vi "HFRR ADV v037.vi"() -> ()   [LabVIEW 2025] (continued)
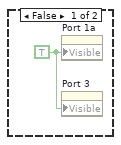
[diagram p5: hidden frame]
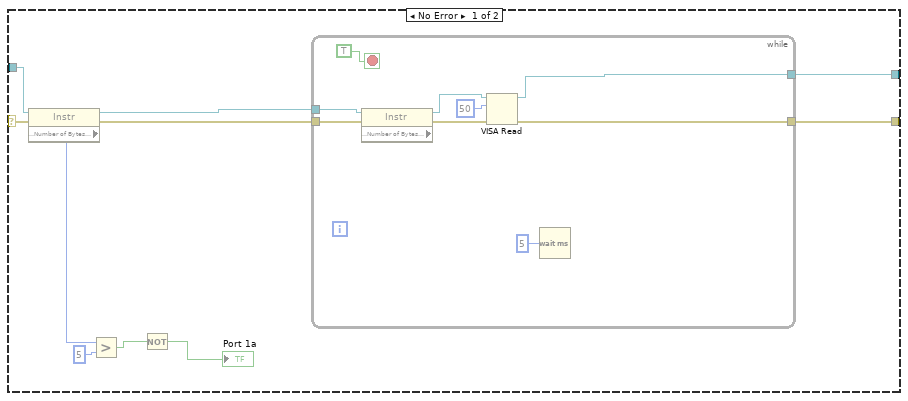
[diagram p6: hidden frame]
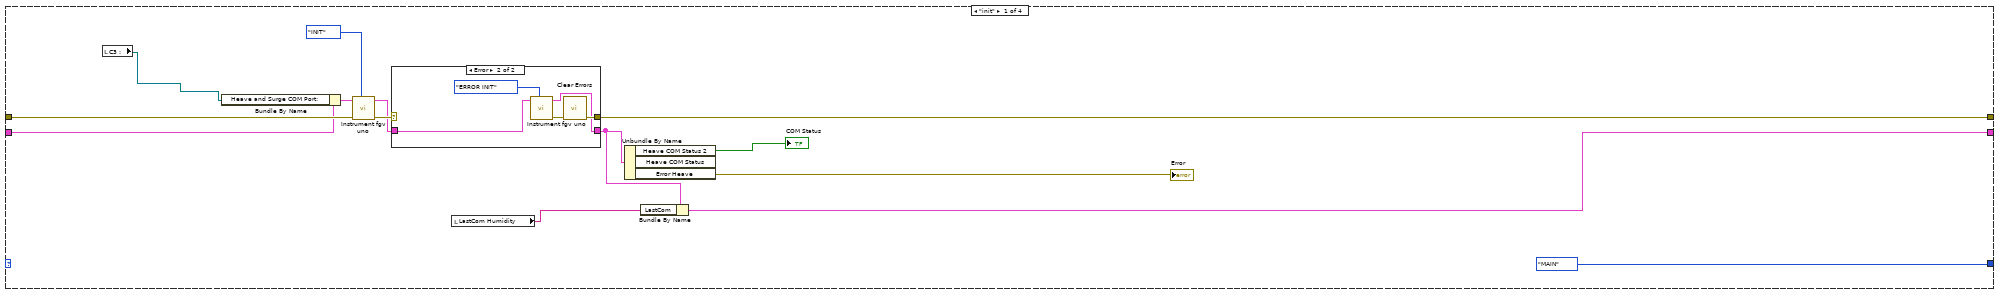
[diagram p8: hidden frame]
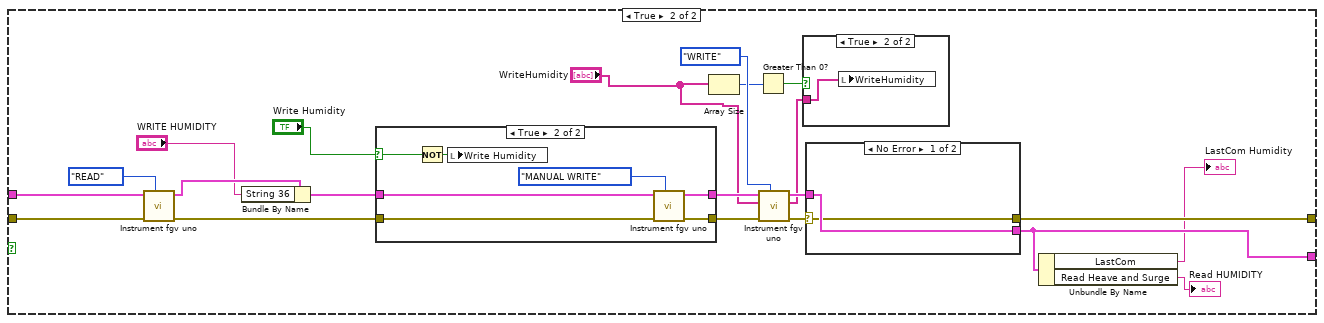
[diagram p11: hidden frame]
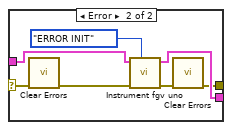
[diagram p13: hidden frame]
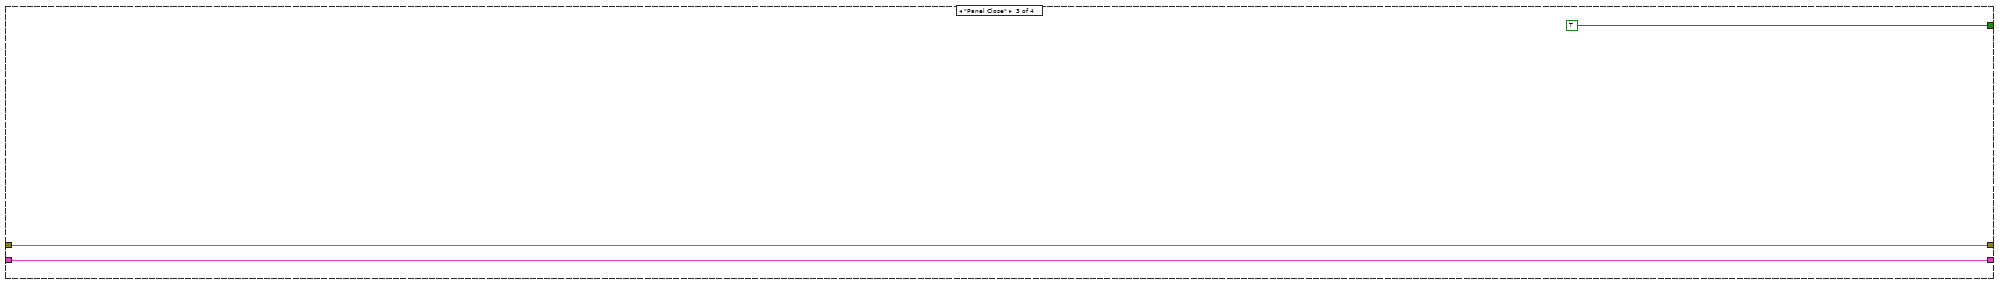
[diagram p15: hidden frame]
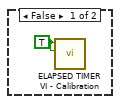
[diagram p19: hidden frame]
        "output Vpp" <- w4040
        n3065 = Number To Fractional String(number=w4040, precision (6)=i16 1) -> (F-format string=w4038:string)  [unwired: 2 in]
        n3066 = Concatenate Strings("DAC;" ("string"), w4038) -> (w4022:string)
        n3067 = local write "Due Write"(w4022) -> ()
        "prev_error" <- w4025
        "integral_accumulator_in" <- w4024
        "prev_vc_cmd" <- w4023
      }
    }
    n3068 = local read "Quit"() -> (w4015:bool)
  }
  n3069 = Or(x=w45, y=w44) -> (x .or. y?=w46:bool)
  n3070 = Or(x=w42, y=w46) -> (x .or. y?=w51:bool)
  n3071 = control-ref of="new picture"() -> ()  [unwired: 1 out]
  n3072 = Or(x=w54, y=w51) -> (x .or. y?=w48:bool)
  n3073 = Or(x=w48, y=w49) -> (x .or. y?=w43:bool)
  n3074 = while {
    tunnel: [w4045] -> w53
    i -> [w4052]
    stop <- w4045 stop-if-true
    n3075 = local read "Quit"() -> (w4045:bool)
    n3076 = Equal To 0?(x=w4052) -> (x = 0?=w4050:bool)
    n3077 = call "Elapsed Time3"("Time Target (s)"=45.0, "Auto Reset"=TRUE) -> ("Time has Elapsed"=w4049:bool)  [unwired: 10 in, 7 out]
    n3078 = Wait (ms)(milliseconds to wait=u32 50) -> ()  [unwired: 1 out]
    n3079 = Or(x=w4049, y=w4050) -> (x .or. y?=w4051:bool)
    n3080 = case shown="True" w4051 {
      frame False {
      }
      frame True {
        n3081 = call <vilib>:"System Exec.vi"("run minimized? (F)"=TRUE, "error in (no error)"="error in (no error)", "command line"="powercfg.exe -change -monitor-timeout-ac 0") -> ("error out"=w4063:errorcluster)  [unwired: 5 in, 3 out]
        n3082 = call <vilib>:"System Exec.vi"("run minimized? (F)"=TRUE, "error in (no error)"=w4063, "command line"="powercfg.exe -change -disk-timeout-ac 0") -> ("error out"=w4062:errorcluster)  [unwired: 5 in, 3 out]
        n3083 = call <vilib>:"System Exec.vi"("run minimized? (F)"=TRUE, "error in (no error)"=w4062, "command line"="powercfg.exe -change -standby-timeout-ac 0") -> ("error out"=w4061:errorcluster)  [unwired: 5 in, 3 out]
        n3084 = call <vilib>:"System Exec.vi"("run minimized? (F)"=TRUE, "error in (no error)"=w4061, "command line"="powercfg.exe -change -hibernate-timeout-ac 0") -> ("error out"=w4060:errorcluster)  [unwired: 5 in, 3 out]
        n3085 = call <vilib>:"Simple Error Handler.vi"("error in (no error)"=w4060) -> ("error out"=w4066:errorcluster)  [unwired: 4 in, 4 out]
        n3086 = call <vilib>:"Clear Errors.vi"("error in (no error)"=w4066) -> ("error out"=→"error out":errorcluster)  [unwired: 5 in, 1 out]
      }
    }
  }
  n3087 = Compound Arithmetic op=OR(w56, w43, w53) -> (w55:bool)
  n3088 = flat-sequence {
    tunnel: w55 -> [_]
    tunnel: [w4068] -> w25
    tunnel: w25 -> [_]
    frame #0 {
      n3089 = call "CLOSE CONNECTION.vi"() -> ("error out"=w4068:errorcluster)  [unwired: 11 in]
    }
    frame #1 {
      n3090 = Quit LabVIEW(quit? (T)=TRUE) -> ()
      n3091 = local write "Quit"(FALSE ("EXIT")) -> ()
    }
  }
  n3092 = property on="Heater Button" class="Bool (strict)"("Visible"=TRUE) -> ()  [unwired: 2 in, 2 out]
  n3093 = while {
    tunnel: [w4075] -> _
    i -> [w4075]
    stop <- w4071 stop-if-true
    # "Langauage selection"
    n3094 = Equal?(x="Lan flag", y=22.0) -> ()  [unwired: 1 out]
    n3095 = disable-structure shown="Disabled" {
      frame Disabled {
        n3096 = stacked-sequence {
          frame #0 {
            n3097 = case shown="\"Russian\"" "Language Selection" {
              tunnel: [0 1] -> w4077
              frame "English", Default {
              }
              frame "Russian" {
              }
            }
            n3098 = for {
              N: 130 -> [_]
              tunnel: "Table" -> [w4086]
              tunnel: w4077 -> [w4085]
              i -> [w4084]
              n3099 = Index Array(array=w4086, index (row)=w4084, index (col)=w4085) -> (element=w4083:string)
              n3100 = case shown="1" w4084 {
                tunnel: w4083 -> [w4087 w4088 _ w4089 w4090 w4091 w4092 w4093 w4094 w4095 w4096 w4097 w4098 w4099 w4100 w4101 w4102 w4103 w4104 w4105 w4106 w4107 w4108 w4109 w4110 w4111 w4112 w4113 w4114 _ _ w4115 w4116 w4117 w4118 w4119 w4120 w4129 w4136 w4143 w4150 w4154 w4157 w4160 w4162 w4164 w4165 w4166 w4167 w4168 w4169 w4170 w4171 w4172 w4173 w4174 w4175 w4176 w4177 w4178 w4179 w4180 w4181 w4182 w4183 w4184 w4185 w4186 w4187 w4188 w4189 w4190 w4191 w4192 w4193 w4194 w4195 w4196 w4197 w4198 w4199 w4200 w4201 w4202 w4203 w4204 w4205 w4206 w4207 w4208 w4209 w4210 w4211 w4212 w4213 w4214 w4215 w4216 w4217 w4218 w4219 w4220 w4221 w4222 w4223 _ w4224 w4225 w4226 w4227 w4228 w4229 w4230 w4231 w4232 w4233 w4234 w4235 w4236 _ w4237 w4238 w4239 w4240 w4241 w4242 _]
                frame 0 {
                  n3101 = local write "S"(w4087) -> ()
                }
                frame 1 {
                  n3102 = local write "S 2"(w4088) -> ()
                }
                frame 2 {
                }
                frame 3 {
                  n3103 = local write "S 4"(w4089) -> ()
                }
                frame 4 {
                  n3104 = property on="FILE" class="Str"("Caption.Text"=w4090) -> ()  [unwired: 2 in, 2 out]
                }
                frame 5 {
                  n3105 = property on="Fuel Discription :" class="Str"("Caption.Text"=w4091) -> ()  [unwired: 2 in, 2 out]
                }
                frame 6 {
                  n3106 = property on="Remarks :" class="Str"("Caption.Text"=w4092) -> ()  [unwired: 2 in, 2 out]
                }
                frame 7 {
                  n3107 = property on="Save & Continue" class="Bool (strict)"("Boolean Text.Text"=w4093) -> ()  [unwired: 2 in, 2 out]
                }
                frame 8 {
                }
                frame 9 {
                  n3108 = property on="Set Hz" class="DigNum (strict)"("Caption.Text"=w4095) -> ()  [unwired: 2 in, 2 out]
                }
                frame 10 {
                }
                frame 11 {
                  n3109 = property on="NORMAL LOAD" class="DigNum (strict)"("Caption.Text"=w4097) -> ()  [unwired: 2 in, 2 out]
                }
                frame 12 {
                }
                frame 13 {
                  n3110 = property on="Set Temp" class="DigNum (strict)"("Caption.Text"=w4099) -> ()  [unwired: 2 in, 2 out]
                }
                frame 14 {
                  n3111 = local write "S 15"(w4100) -> ()
                }
                frame 15 {
                  n3112 = property on="Set Rh" class="DigNum (strict)"("Caption.Text"=w4101) -> ()  [unwired: 2 in, 2 out]
                }
                frame 16 {
                }
                frame 17 {
                  n3113 = local write "S 18"(w4103) -> ()
                }
                frame 18 {
                  "String 17" <- w4104
                }
                frame 19 {
                  n3114 = property on="test time" class="DigNum (strict)"("Caption.Text"=w4105) -> ()  [unwired: 2 in, 2 out]
                }
                frame 20 {
                  "String 18" <- w4106
                  "String 22" <- w4106
                }
                frame 21 {
                  n3115 = property on="Elapsed time" class="DigNum (strict)"("Caption.Text"=w4107) -> ()  [unwired: 2 in, 2 out]
                }
                frame 22 {
                  n3116 = property on="Samplingtime 2" class="DigNum (strict)"("Caption.Text"=w4108) -> ()  [unwired: 2 in, 2 out]
                }
                frame 23 {
                  "String 21" <- w4109
                }
                frame 24 {
                  n3117 = property on="Countdown" class="DigNum (strict)"("Caption.Text"=w4110) -> ()  [unwired: 2 in, 2 out]
                }
                frame 25 {
                  n3118 = property on="Countdown 2" class="DigNum (strict)"("Caption.Text"=w4111) -> ()  [unwired: 2 in, 2 out]
                }
                frame 26 {
                  n3119 = property on="Engage" class="Bool (strict)"("Boolean Text.Text"=w4112) -> ()  [unwired: 2 in, 2 out]
                }
                frame 27 {
                  n3120 = property on="Boolean  4" class="Bool (strict)"("Boolean Text.Text"=w4113) -> ()  [unwired: 2 in, 2 out]
                }
                frame 28 {
                  n3121 = property on="Test \nStatus" class="Bool (strict)"("Boolean Text.Text"=w4114) -> ()  [unwired: 2 in, 2 out]
                }
                frame 29 {
                }
                frame 30 {
                }
                frame 31 {
                }
                frame 32 {
                  n3122 = property on="RSTCOF" class="Bool"("Boolean Text.Text"=w4116) -> ()  [unwired: 2 in, 2 out]
                  n3123 = property on="RST FF" class="Bool"("Boolean Text.Text"=w4116) -> ()  [unwired: 2 in, 2 out]
                  n3124 = property on="RST TEMP" class="Bool"("Boolean Text.Text"=w4116) -> ()  [unwired: 2 in, 2 out]
                  n3125 = property on="RSTV1 3" class="Bool"("Boolean Text.Text"=w4116) -> ()  [unwired: 2 in, 2 out]
                  n3126 = property on="rstv2" class="Bool"("Boolean Text.Text"=w4116) -> ()  [unwired: 2 in, 2 out]
                  n3127 = property on="RSTV1 2" class="Bool"("Boolean Text.Text"=w4116) -> ()  [unwired: 2 in, 2 out]
                  n3128 = property on="RST CP" class="Bool"("Boolean Text.Text"=w4116) -> ()  [unwired: 2 in, 2 out]
                }
                frame 33 {
                  "S 61" <- w4117
                }
                frame 34 {
                  "String 23" <- w4118
                }
                frame 35 {
                  n3129 = property on="Rh Before" class="DigNum (strict)"("Caption.Text"=w4119) -> ()  [unwired: 2 in, 2 out]
                }
                frame 36 {
                  n3130 = Match Pattern(string=w4120, regular expression=",") -> (before substring=→"bs":string, after substring=→"as":string)  [unwired: 1 in, 2 out]
                  n3131 = property on="Rh After" class="DigNum (strict)"("Caption.Text"=w4120) -> ()  [unwired: 2 in, 2 out]
                }
                frame 37 {
                  n3132 = Match Pattern(string=w4129, regular expression=",") -> (before substring=w4128:string, after substring=w4127:string)  [unwired: 1 in, 2 out]
                  "bs" <- w4128
                  "as" <- w4127
                  n3133 = Concatenate Strings(w4128, w4127) -> (w4124:string)
                  n3134 = property on="Humidity before test 2" class="DigNum (strict)"("Caption.Text"=w4124) -> ()  [unwired: 2 in, 2 out]
                  n3135 = Concatenate Strings(w4124, "=" ("string")) -> (w4125:string)
                  n3136 = local write "S 38"(w4125) -> ()
                }
                frame 38 {
                  n3137 = Match Pattern(string=w4136, regular expression=",") -> (before substring=w4135:string, after substring=w4134:string)  [unwired: 1 in, 2 out]
                  "bs" <- w4135
                  "as" <- w4134
                  n3138 = Concatenate Strings(w4135, w4134) -> (w4131:string)
                  n3139 = property on="Humidity after test 2" class="DigNum (strict)"("Caption.Text"=w4131) -> ()  [unwired: 2 in, 2 out]
                  n3140 = Concatenate Strings(w4131, "=" ("string")) -> (w4133:string)
                  n3141 = local write "S 39"(w4133) -> ()
                }
                frame 39 {
                  n3142 = Match Pattern(string=w4143, regular expression=",") -> (before substring=w4142:string, after substring=w4141:string)  [unwired: 1 in, 2 out]
                  "bs" <- w4142
                  "as" <- w4141
                  n3143 = Concatenate Strings(w4142, w4141) -> (w4138:string)
                  n3144 = property on="Temperature before test 2" class="DigNum (strict)"("Caption.Text"=w4138) -> ()  [unwired: 2 in, 2 out]
                  n3145 = Concatenate Strings(w4138, "=" ("string")) -> (→"String 34":string)
                }
                frame 40 {
                  n3146 = Match Pattern(string=w4150, regular expression=",") -> (before substring=w4149:string, after substring=w4148:string)  [unwired: 1 in, 2 out]
                  "bs" <- w4149
                  "as" <- w4148
                  n3147 = Concatenate Strings(w4149, w4148) -> (w4145:string)
                  n3148 = property on="Temperature after test 2" class="DigNum (strict)"("Caption.Text"=w4145) -> ()  [unwired: 2 in, 2 out]
                  n3149 = Concatenate Strings(w4145, "=" ("string")) -> (→"String 35":string)
                  n3150 = property on="Temperature after test" class="DigNum (strict)"("Caption.Text"=w4145) -> ()  [unwired: 2 in, 2 out]
                }
                frame 41 {
                  n3151 = property on="AVP 2" class="DigNum (strict)"("Caption.Text"=w4154) -> ()  [unwired: 2 in, 2 out]
                  n3152 = Concatenate Strings(w4154, "=" ("string")) -> (→"String 36":string)
                }
                frame 42 {
                  n3153 = property on="MWSD 2" class="DigNum (strict)"("Caption.Text"=w4157) -> ()  [unwired: 2 in, 2 out]
                  n3154 = Concatenate Strings(w4157, "=" ("string")) -> (→"String 37":string)
                }
                frame 43 {
                  n3155 = property on="HCF 2" class="DigNum (strict)"("Caption.Text"=w4160) -> ()  [unwired: 2 in, 2 out]
                  n3156 = Concatenate Strings(w4160, "=" ("string")) -> (→"String 38":string)
                }
                frame 44 {
                  n3157 = Concatenate Strings(w4162, "=" ("string")) -> (→"String 39":string)
                  n3158 = property on="WS1.4 2" class="DigNum (strict)"("Caption.Text"=w4162) -> ()  [unwired: 2 in, 2 out]
                }
                frame 45 {
                }
                frame 46 {
                  n3159 = local write "S 47"(w4165) -> ()
                }
                frame 47 {
                  n3160 = local write "S 48"(w4166) -> ()
                }
                frame 48 {
                  n3161 = local write "S 49"(w4167) -> ()
                }
                frame 49 {
                  n3162 = local write "S 50"(w4168) -> ()
                }
                frame 50 {
                  n3163 = local write "S 51"(w4169) -> ()
                }
                frame 51 {
                  n3164 = local write "S 52"(w4170) -> ()
                }
                frame 52 {
                  n3165 = local write "S 53"(w4171) -> ()
                }
                frame 53 {
                  n3166 = local write "S 54"(w4172) -> ()
                }
                frame 54 {
                  n3167 = local write "S 55"(w4173) -> ()
                }
                frame 55 {
                  n3168 = local write "S 56"(w4174) -> ()
                }
                frame 56 {
                  n3169 = local write "S 57"(w4175) -> ()
                }
                frame 57 {
                  n3170 = local write "S 58"(w4176) -> ()
                }
                frame 58 {
                  n3171 = local write "S 59"(w4177) -> ()
                }
                frame 59 {
                  n3172 = local write "S 60"(w4178) -> ()
                }
                frame 60 {
                  n3173 = local write "S 62"(w4179) -> ()
                }
                frame 61 {
                  n3174 = local write "S 63"(w4180) -> ()
                }
                frame 62 {
                  n3175 = local write "S 64"(w4181) -> ()
                }
                frame 63 {
                  n3176 = local write "S 65"(w4182) -> ()
                }
                frame 64 {
                  n3177 = local write "S 66"(w4183) -> ()
                }
                frame 65 {
                  n3178 = local write "S 67"(w4184) -> ()
                }
                frame 66 {
                  n3179 = local write "S 68"(w4185) -> ()
                }
                frame 67 {
                  n3180 = local write "S 69"(w4186) -> ()
                }
                frame 68 {
                  n3181 = local write "S 70"(w4187) -> ()
                }
                frame 69 {
                  n3182 = local write "S 71"(w4188) -> ()
                }
                frame 70 {
                  n3183 = local write "S 72"(w4189) -> ()
                }
                frame 71 {
                  n3184 = local write "S 73"(w4190) -> ()
                }
                frame 72 {
                  n3185 = local write "S 74"(w4191) -> ()
                }
                frame 73 {
                  n3186 = local write "S 75"(w4192) -> ()
                }
                frame 74 {
                  n3187 = local write "S 76"(w4193) -> ()
                }
                frame 75 {
                  n3188 = local write "S 77"(w4194) -> ()
                }
                frame 76 {
                  n3189 = local write "S 78"(w4195) -> ()
                }
                frame 77 {
                  n3190 = local write "S 79"(w4196) -> ()
                }
                frame 79 {
                  n3191 = property on="Sample Temperature ( °C )" class="XYGraph (strict)"("Y Scale.Name Label.Text"=w4197) -> ()  [unwired: 2 in, 2 out]
                }
                frame 80 {
                  n3192 = local write "S 81"(w4198) -> ()
                  n3193 = property on="Humidity ( %RH )" class="XYGraph (strict)"("Y Scale.Name Label.Text"=w4198) -> ()  [unwired: 2 in, 2 out]
                }
                frame 78 {
                  n3194 = property on="Air Temperature  ( °C )" class="XYGraph (strict)"("X Scale.Name Label.Text"=w4199) -> ()  [unwired: 2 in, 2 out]
                  n3195 = property on="Humidity ( %RH )" class="XYGraph (strict)"("X Scale.Name Label.Text"=w4199) -> ()  [unwired: 2 in, 2 out]
                  n3196 = property on="Sample Temperature ( °C )" class="XYGraph (strict)"("X Scale.Name Label.Text"=w4199) -> ()  [unwired: 2 in, 2 out]
                  n3197 = property on="Coefficient Of Friction" class="XYGraph (strict)"("X Scale.Name Label.Text"=w4199) -> ()  [unwired: 2 in, 2 out]
                }
                frame 81 {
                  n3198 = property on="Air Temperature  ( °C )" class="XYGraph (strict)"("Y Scale.Name Label.Text"=w4200) -> ()  [unwired: 2 in, 2 out]
                }
                frame 82 {
                  n3199 = local write "S 84"(w4201) -> ()
                }
                frame 83 {
                  n3200 = local write "S 85"(w4202) -> ()
                }
                frame 84 {
                  n3201 = local write "S 86"(w4203) -> ()
                }
                frame 85 {
                  n3202 = local write "S 87"(w4204) -> ()
                }
                frame 86 {
                  n3203 = local write "S 88"(w4205) -> ()
                }
                frame 87 {
                }
                frame 88 {
                  n3204 = local write "S 90"(w4207) -> ()
                }
                frame 89 {
                  n3205 = local write "S 91"(w4208) -> ()
                }
                frame 90 {
                  n3206 = local write "S 92"(w4209) -> ()
                }
                frame 91 {
                  n3207 = local write "S 93"(w4210) -> ()
                }
                frame 92 {
                  n3208 = local write "S 94"(w4211) -> ()
                }
                frame 93 {
                  n3209 = local write "S 95"(w4212) -> ()
                }
                frame 94 {
                  n3210 = local write "S 96"(w4213) -> ()
                }
                frame 95 {
                  n3211 = local write "S 97"(w4214) -> ()
                }
                frame 96 {
                  n3212 = local write "S 98"(w4215) -> ()
                }
                frame 97 {
                  n3213 = local write "S 99"(w4216) -> ()
                }
                frame 98 {
                  n3214 = local write "S 100"(w4217) -> ()
                }
                frame 99 {
                  n3215 = local write "S 101"(w4218) -> ()
                }
                frame 100 {
                  n3216 = local write "S 102"(w4219) -> ()
                }
                frame 101 {
                  n3217 = local write "S 103"(w4220) -> ()
                }
                frame 102 {
                  n3218 = local write "S 104"(w4221) -> ()
                }
                frame 103 {
                  n3219 = local write "S 105"(w4222) -> ()
                }
                frame 104 {
                  n3220 = local write "S 106"(w4223) -> ()
                }
                frame 105 {
                }
                frame 106 {
                  n3221 = property on="OK Button 17" class="Bool (strict)"("Boolean Text.Text"=w4224) -> ()  [unwired: 2 in, 2 out]
                }
                frame 107 {
                  n3222 = property on="OK Button 16" class="Bool (strict)"("Boolean Text.Text"=w4225) -> ()  [unwired: 2 in, 2 out]
                }
                frame 108 {
                  n3223 = property on="TITTLE" class="Str"("Caption.Text"=w4226) -> ()  [unwired: 2 in, 2 out]
                }
                frame 109 {
                  "String 30" <- w4227
                }
                frame 110 {
                  n3224 = property on="Test Date" class="Str"("Caption.Text"=w4228) -> ()  [unwired: 2 in, 2 out]
                  "String 31" <- w4228
                }
                frame 111 {
                  n3225 = property on="Sample ID" class="Str"("Caption.Text"=w4229) -> ()  [unwired: 2 in, 2 out]
                  "String 32" <- w4229
                }
                frame 112 {
                  n3226 = property on="Tested by" class="Str"("Caption.Text"=w4230) -> ()  [unwired: 2 in, 2 out]
                  "String 33" <- w4230
                }
                frame 113 {
                  n3227 = property on="System Configured Printers 2" class="Arr (strict)"("Caption.Text"=w4231) -> ()  [unwired: 2 in, 2 out]
                }
                frame 114 {
                  n3228 = property on="Selected Printer" class="Str"("Caption.Text"=w4232) -> ()  [unwired: 2 in, 2 out]
                }
                frame 115 {
                  n3229 = property on="Select Printer 3" class="DigNum (strict)"("Caption.Text"=w4233) -> ()  [unwired: 2 in, 2 out]
                }
                frame 116 {
                  n3230 = property on="Print" class="Bool (strict)"("Boolean Text.Text"=w4234) -> ()  [unwired: 2 in, 2 out]
                }
                frame 117 {
                  "String 41" <- w4235
                }
                frame 118 {
                  n3231 = property on="tested by" class="Str"("Caption.Text"=w4236) -> ()  [unwired: 2 in, 2 out]
                }
                frame 119 {
                }
                frame 120 {
                  n3232 = property on="Export" class="Bool (strict)"("Boolean Text.Text"=w4237) -> ()  [unwired: 2 in, 2 out]
                }
                frame 121 {
                }
                frame 122 {
                }
                frame 123 {
                  n3233 = property on="Select File Type" class="Enum (strict)"("Caption.Text"=w4240) -> ()  [unwired: 2 in, 2 out]
                }
                frame 124 {
                  n3234 = property on="s.NO" class="Str"("Caption.Text"=w4241) -> ()  [unwired: 2 in, 2 out]
                  "String 45" <- w4241
                }
                frame 125 {
                  n3235 = property on="trip1 8" class="Bool (strict)"("Boolean Text.Text"=w4242) -> ()  [unwired: 2 in, 2 out]
                }
                frame 126, Default {
                }
              }
            }
          }
          frame #1 {
            w4250 = TRUE ("Visible")
            n3236 = local read "S 91"() -> (w4267:string)
            n3237 = local read "S 90"() -> (w4266:string)
            n3238 = local read "S 88"() -> (w4265:string)
            n3239 = property on="File Path" class="Path"("Caption.Text"=w4266) -> ()  [unwired: 2 in, 2 out]
            n3240 = local read "S 71"() -> (w4260:string)
            n3241 = local read "S 86"() -> (w4262:string)
            n3242 = local read "S 85"() -> (w4263:string)
            n3243 = local read "S 87"() -> (w4261:string)
            n3244 = local read "S 84"() -> (w4264:string)
            n3245 = local read "S 103"() -> (w4249:string)
            n3246 = local read "S 104"() -> (w4248:string)
            n3247 = property on="Password" class="Str"("Caption.Text"=w4263) -> ()  [unwired: 2 in, 2 out]
            n3248 = property on="EDIT" class="Bool (strict)"("Boolean Text.Text"=w4260) -> ()  [unwired: 2 in, 2 out]
            n3249 = property on="SAVE" class="Bool (strict)"("Boolean Text.Text"=w4264) -> ()  [unwired: 2 in, 2 out]
            n3250 = Build Array(w4249, w4248) -> (w4247:string[])
            n3251 = property on="Heater Button" class="Bool (strict)"("Strings [4]"=w4247) -> ()  [unwired: 2 in, 2 out]
            n3252 = local read "S 92"() -> (w4259:string)
            n3253 = local read "S 93"() -> (w4258:string)
            n3254 = local read "S 105"() -> (w4245:string)
            n3255 = local read "S 106"() -> (w4244:string)
            n3256 = Build Array(w4259, w4258) -> ()  [unwired: 1 out]
            n3257 = Build Array(w4245, w4244) -> (w4246:string[])
            n3258 = local read "S 95"() -> (w4256:string)
            n3259 = local read "S 94"() -> (w4257:string)
            n3260 = local read "bs"() -> (w4272:string)
            n3261 = local read "as"() -> (w4273:string)
            n3262 = property on="Humidity" class="Bool (strict)"("Strings [4]"=w4246) -> ()  [unwired: 2 in, 2 out]
            n3263 = Concatenate Strings(w4272, "\r", w4273) -> ()  [unwired: 1 out]
            n3264 = property on="Rh After" class="DigNum (strict)"("Caption.Size to Text?"=TRUE ("Caption.Size to Text")) -> ()  [unwired: 2 in, 2 out]
            n3265 = local read "S 48"() -> (w4296:string)
            n3266 = local read "S 50"() -> (w4294:string)
            n3267 = local read "S 51"() -> (w4293:string)
            n3268 = local read "S 49"() -> (w4295:string)
            n3269 = local read "S 52"() -> (w4292:string)
            n3270 = local read "as"() -> (w4277:string)
            n3271 = local read "bs"() -> (w4278:string)
            n3272 = local read "S 56"() -> (w4291:string)
            n3273 = local read "S 57"() -> (w4290:string)
            n3274 = local read "S 58"() -> (w4289:string)
            n3275 = local read "S 59"() -> (w4288:string)
            n3276 = property on="OPEN" class="Bool (strict)"("Boolean Text.Text"=w4292) -> ()  [unwired: 2 in, 2 out]
            n3277 = property on="OPEN 1" class="Bool (strict)"("Boolean Text.Text"=w4296) -> ()  [unwired: 2 in, 2 out]
            n3278 = property on="OPEN 2" class="Bool (strict)"("Boolean Text.Text"=w4295) -> ()  [unwired: 2 in, 2 out]
            n3279 = property on="OPEN 3" class="Bool (strict)"("Boolean Text.Text"=w4294) -> ()  [unwired: 2 in, 2 out]
            n3280 = property on="OPEN 4" class="Bool (strict)"("Boolean Text.Text"=w4293) -> ()  [unwired: 2 in, 2 out]
            n3281 = Concatenate Strings(w4278, "\r", w4277) -> ()  [unwired: 1 out]
            n3282 = local read "S 102"() -> (w4251:string)
            n3283 = property on="КОФ1" class="DigNum (strict)"("Caption.Text"=w4291) -> ()  [unwired: 2 in, 2 out]
            n3284 = local read "S 98"() -> (w4255:string)
            n3285 = local read "S 99"() -> (w4254:string)
            n3286 = local read "S 100"() -> (w4253:string)
            n3287 = local read "S 101"() -> (w4252:string)
            n3288 = property on="КОФ2" class="DigNum (strict)"("Caption.Text"=w4290) -> ()  [unwired: 2 in, 2 out]
            n3289 = property on="КОФ3" class="DigNum (strict)"("Caption.Text"=w4289) -> ()  [unwired: 2 in, 2 out]
            n3290 = property on="КОФ4" class="DigNum (strict)"("Caption.Text"=w4288) -> ()  [unwired: 2 in, 2 out]
            n3291 = local read "bs"() -> (w4276:string)
            n3292 = local read "as"() -> (w4275:string)
            n3293 = local read "S 60"() -> (w4287:string)
            n3294 = local read "S 54"() -> (w4297:string)
            n3295 = Concatenate Strings(w4276, "\r", w4275) -> ()  [unwired: 1 out]
            n3296 = Concatenate Strings(w4297, w4287) -> ()  [unwired: 1 out]
            n3297 = local read "S 77"() -> (→"String 43":string)
            n3298 = local read "S 76"() -> (w4270:string)
            n3299 = local read "S 78"() -> (w4269:string)
            n3300 = local read "S 71"() -> (w4281:string)
            n3301 = local read "S 66"() -> (w4286:string)
            n3302 = local read "S 67"() -> (w4285:string)
            n3303 = local read "S 68"() -> (w4284:string)
            n3304 = local read "S 69"() -> (w4283:string)
            n3305 = local read "S 70"() -> (w4282:string)
            n3306 = property on="AIR TEMP" class="DigNum (strict)"("Caption.Text"=w4269) -> ()  [unwired: 2 in, 2 out]
            n3307 = property on="Set Strk" class="DigNum (strict)"("Caption.Text"=w4270) -> ()  [unwired: 2 in, 2 out]
            n3308 = property on="SPEED OUT:" class="DigNum (strict)"("Caption.Text"=w4284) -> ()  [unwired: 2 in, 2 out]
            n3309 = property on="EDIT" class="Bool (strict)"("Boolean Text.Text"=w4281) -> ()  [unwired: 2 in, 2 out]
            n3310 = local read "S 79"() -> (w4268:string)
          }
          frame #2 {
          }
        }
        n3311 = local write "Lan flag"(10.0 ("Lan flag")) -> ()
      }
      frame Enabled {
      }
    }
    n3312 = Wait (ms)(milliseconds to wait=u32 2000) -> ()  [unwired: 1 out]
    n3313 = local read "Quit"() -> (w4071:bool)
  }
  n3314 = while {
    shift-right: [w4303] -> _
    shift-left: _ -> [w4304]
    shift-right: [w4301] -> _
    shift-left: T18 {"Read Heave and Surge"="", "Bytes at Heave Port"=0.0, "Heave and Surge COM Port:"="COM9", "Com Port 2"="COM7", "Residual Due"="", "Heave COM Status 2"=TRUE, "Heave COM Status"=TRUE, "Port 2"=TRUE, "Sway PPR"=6400.0, "Surge PPR"=6400.0, "Heave PPR"=6400.0, "Sway Pitch"=2.0, "Surge Pitch"=3.0, "Heave Pitch"=4.0, "Sway Pulses/mm"=320.0, "Surge Pulses/mm"=1600.0, "Heave Pulses/mm"=1600.0, "inner loop"=0.0, "Read Heave and Surge 2"="", "String 36"="", "Write S"=FALSE, "WriteCC1"=[""], "Heave COM Loop"=0, "LastCom"="", "EXIT"=FALSE, "Error Heave"={"status"=TRUE, "code"=-1073807343, "source"=""}} -> [w4300]
    shift-right: [w4298] -> _
    shift-left: enum16{"init", "MAIN", "Panel Close"}."init" -> [w4299]
    stop <- w4302 stop-if-true
    # "HUMIDITY LOOP LOGIC"
    n3315 = case shown="\"MAIN\"" w4299 {
      tunnel: w4304 -> [w4318 w4342 w4406 w4408]
      tunnel: [w4313 w4329 w4406 w4408] -> w4303
      tunnel: [_ _ TRUE _] -> w4302
      tunnel: [w4310 w4327 w4404 w4407] -> w4301
      tunnel: w4300 -> [w4315 w4341 w4404 w4407]
      tunnel: [enum16{"init", "MAIN", "Panel Close"}."MAIN" w4336 _ _] -> w4298
      frame "init" {
        n3316 = local read "C3 :"() -> (w4305:refnum<visa-resource-name>)
        n3317 = Bundle By Name(cluster=w4315, "Heave and Surge COM Port:"=w4305) -> (w4314:T18)
        n3318 = call "Instrument fgv uno.vi"("Enum"=T32."INIT", "error in (no error) 2"=w4318, "INPUT"=w4314) -> ("error"=w4316:errorcluster, "output"=w4312:T18)  [unwired: 6 in, 1 out]
        n3319 = case shown="Error" w4316 {
          selector: w4316 -> [w4320 _]
          tunnel: [w4320 w4324] -> w4313
          tunnel: w4312 -> [w4319 w4322]
          tunnel: [w4319 w4321] -> w4311
          frame No Error {
          }
          frame Error {
            n3320 = call "Instrument fgv uno.vi"("Enum"=T32."ERROR INIT", "INPUT"=w4322) -> ("error"=w4325:errorcluster, "output"=w4321:T18)  [unwired: 7 in, 1 out]
            n3321 = call <vilib>:"Clear Errors.vi"("error in (no error)"=w4325) -> ("error out"=w4324:errorcluster)  [unwired: 5 in, 1 out]
          }
        }
        n3322 = local read "LastCom Humidity"() -> (w4308:string)
        n3323 = Unbundle By Name(w4311) -> ("Heave COM Status 2"=→"COM Status":bool, "Error Heave"=→"Error":errorcluster)  [unwired: 1 out]
        n3324 = Bundle By Name(cluster=w4311, "LastCom"=w4308) -> (w4310:T18)
      }
      frame "MAIN" {
        n3325 = Unbundle By Name(w4341) -> ("Com Port 2"=w4331:refnum<visa-resource-name>)
        n3326 = local read "C3 :"() -> (w4332:refnum<visa-resource-name>)
        n3327 = local write "COM Port Humidity :"(w4331) -> ()
        n3328 = Bundle By Name(cluster=w4341, "Heave and Surge COM Port:"=w4332) -> (w4340:T18)
        n3329 = Equal?(x=w4331, y=w4332) -> (x = y?=w4345:bool)
        n3330 = case shown="False" w4345 {
          tunnel: [w4360 w4377] -> w4330
          tunnel: w4342 -> [w4361 w4383]
          tunnel: w4340 -> [w4359 w4381]
          tunnel: [w4358 w4376] -> w4328
          frame False {
            n3331 = call <vilib>:"Clear Errors.vi"("error in (no error)"=w4361) -> ("error out"=w4357:errorcluster)  [unwired: 5 in, 1 out]
            n3332 = call "Instrument fgv uno.vi"("Enum"=T32."ERROR INIT", "error in (no error) 2"=w4357, "INPUT"=w4359) -> ("error"=w4363:errorcluster, "output"=w4358:T18)  [unwired: 6 in, 1 out]
            n3333 = call <vilib>:"Clear Errors.vi"("error in (no error)"=w4363) -> ("error out"=w4360:errorcluster)  [unwired: 5 in, 1 out]
          }
          frame True {
            n3334 = call "Instrument fgv uno.vi"("Enum"=T32."READ", "error in (no error) 2"=w4383, "INPUT"=w4381) -> ("error"=w4382:errorcluster, "output"=w4375:T18)  [unwired: 6 in, 1 out]
            n3335 = Bundle By Name(cluster=w4375, "String 36"="WRITE HUMIDITY") -> (w4374:T18)
            n3336 = case shown="True" "Write Humidity" {
              selector: "Write Humidity" -> [_ w4403]
              tunnel: w4382 -> [w4396 w4402]
              tunnel: [w4396 w4401] -> w4372
              tunnel: w4374 -> [w4395 w4399]
              tunnel: [w4395 w4398] -> w4371
              frame False {
              }
              frame True {
                n3337 = Not(x=w4403) -> (.not. x?=w4397:bool)
                n3338 = local write "Write Humidity"(w4397) -> ()
                n3339 = call "Instrument fgv uno.vi"("Enum"=T32."MANUAL WRITE", "error in (no error) 2"=w4402, "INPUT"=w4399) -> ("error"=w4401:errorcluster, "output"=w4398:T18)  [unwired: 6 in, 1 out]
              }
            }
            n3340 = Array Size(array="WriteHumidity") -> (size(s)=w4369:i32)
            n3341 = Greater Than 0?(x=w4369) -> (x > 0?=w4368:bool)
            n3342 = call "Instrument fgv uno.vi"("Enum"=T32."WRITE", "error in (no error) 2"=w4372, "WriteCC1"="WriteHumidity", "INPUT"=w4371) -> ("error"=w4379:errorcluster, "WriteCC1 2"=w4370:string[], "output"=w4378:T18)  [unwired: 5 in]
            n3343 = case shown="True" w4368 {
              tunnel: w4370 -> [_ w4385]
              frame False {
              }
              frame True {
                n3344 = local write "WriteHumidity"(w4385) -> ()
              }
            }
            n3345 = case shown="No Error" w4379 {
              selector: w4379 -> [w4386 w4389]
              tunnel: w4378 -> [w4387 w4394]
              tunnel: [w4387 w4393] -> w4376
              tunnel: [w4386 w4391] -> w4377
              frame No Error {
              }
              frame Error {
                n3346 = call <vilib>:"Clear Errors.vi"("error in (no error)"=w4389) -> ("error out"=w4388:errorcluster)  [unwired: 5 in, 1 out]
                n3347 = call "Instrument fgv uno.vi"("Enum"=T32."ERROR INIT", "error in (no error) 2"=w4388, "INPUT"=w4394) -> ("error"=w4392:errorcluster, "output"=w4393:T18)  [unwired: 6 in, 1 out]
                n3348 = call <vilib>:"Clear Errors.vi"("error in (no error)"=w4392) -> ("error out"=w4391:errorcluster)  [unwired: 5 in, 1 out]
              }
            }
            n3349 = Unbundle By Name(w4376) -> ("LastCom"=→"LastCom Humidity":string, "Read Heave and Surge"=→"Read HUMIDITY":string)
          }
        }
        n3350 = Unbundle By Name(w4328) -> ("Heave COM Status 2"=w4344:bool, "Error Heave"=w4333:errorcluster, "Bytes at Heave Port"=→"Bytes at Humidity Port  2":dbl)  [unwired: 1 out]
        n3351 = Unbundle By Name(w4333) -> ("status"=→"Humidity Port":bool)
        n3352 = Not(x=w4344) -> (.not. x?=w4334:bool)
        n3353 = local write "Error"(w4333) -> ()
        n3354 = local read "Quit"() -> (w4337:bool)
        n3355 = local write "COM Status"(w4334) -> ()
        n3356 = Select(t=enum16{"init", "MAIN", "Panel Close"}."Panel Close", s=w4337, f=enum16{"init", "MAIN", "Panel Close"}."MAIN") -> (s? t:f=w4336:enum16{"init", "MAIN", "Panel Close"})
        n3357 = local read "Humidity"() -> (w4326:bool)
        n3358 = case shown="True" w4326 {
          selector: w4326 -> [_ w4348]
          tunnel: w4330 -> [w4346 w4353]
          tunnel: [w4346 w4352] -> w4329
          tunnel: w4328 -> [w4347 w4351]
          tunnel: [w4347 w4350] -> w4327
          frame False {
          }
          frame True {
            n3359 = Not(x=w4348) -> (.not. x?=→"Humidity":bool)
            n3360 = call <vilib>:"Clear Errors.vi"("error in (no error)"=w4353) -> ("error out"=w4356:errorcluster)  [unwired: 5 in, 1 out]
            n3361 = call "Instrument fgv uno.vi"("Enum"=T32."ERROR INIT", "error in (no error) 2"=w4356, "INPUT"=w4351) -> ("error"=w4354:errorcluster, "output"=w4350:T18)  [unwired: 6 in, 1 out]
            n3362 = call <vilib>:"Clear Errors.vi"("error in (no error)"=w4354) -> ("error out"=w4352:errorcluster)  [unwired: 5 in, 1 out]
          }
        }
      }
      frame "Panel Close" {
      }
      frame Default {
      }
    }
  }
  n3363 = while {
    stop <- w4410 stop-if-true
    n3364 = call <vilib>:"High Resolution Polling Wait.vi"("seconds to wait"=0.05) -> ()  [unwired: 10 in, 1 out]
    n3365 = disable-structure shown="Enabled" {
      frame Disabled {
        n3366 = local read "Read HUMIDITY"() -> (w4411:string)
        n3367 = Spreadsheet String To Array(delimiter (Tab)=",", format string="", spreadsheet string=w4411, array type (2D Dbl)=string[] []) -> (array=w4430:string[])
        n3368 = for {
          tunnel: w4430 -> [w4439] mode=indexing
          tunnel: string[] ["STATE;", "SET;", "RH;", "T;", "AMB_RH;", "AMB_T;", "PUMP;", "FAN_IN;", "FAN_OUT;", "DEHUM;", "CURRENT;", "STALL;"] -> [w4438] mode=indexing
          tunnel: [w4437] -> w4429 mode=indexing
          n3369 = Match Pattern(string=w4439, regular expression=w4438) -> (after substring=w4437:string)  [unwired: 1 in, 3 out]
        }
        n3370 = Index Array(array=w4429) -> (element #1=→"STATE :":string, element #2=→"SET :":string, element #3=w4419:string, element #4=→"T :":string, element #5=w4417:string, element #6=→"AMB_T :":string, element #7=→"PUMP :":string, element #8=→"FAN_IN :":string, element #9=→"FAN_OUT :":string, element #10=→"DEHUM :":string, element #11=→"CURRENT :":string, element #12=→"STALL :":string)  [unwired: 12 in]
        "RH :" <- w4419
        "AMB_RH :" <- w4417
        n3371 = Fract/Exp String To Number(string=w4419) -> (number=w4412:dbl)  [unwired: 3 in, 1 out]
        n3372 = Fract/Exp String To Number(string=w4417) -> (number=w4416:dbl)  [unwired: 3 in, 1 out]
        n3373 = local write "Ambient Humidity :"(w4416) -> ()
        n3374 = Equal?(x=w4412, y=0.0) -> (x = y?=w4414:bool)
        n3375 = case shown="True" w4414 {
          tunnel: [w4435 w4436] -> w4413
          tunnel: w4412 -> [w4435 _]
          frame False {
            (unwired) 0.0
            "Humidity temp" <- w4435
          }
          frame True {
            n3376 = local read "Humidity temp"() -> (w4436:dbl)
          }
        }
        "RH Numeric:" <- w4413
      }
      frame Enabled {
        n3377 = local read "Read HUMIDITY"() -> (w4460:string)
        n3378 = Spreadsheet String To Array(delimiter (Tab)=",", format string="", spreadsheet string=w4460, array type (2D Dbl)=dbl[] []) -> (array=w4456:dbl[])
        n3379 = Index Array(array=w4456) -> (element #1=→"STATE :":dbl, element #2=→"SET :":dbl, element #3=w4440:dbl, element #4=→"RH :":dbl, element #5=→"T :":dbl, element #6=→"AMB_RH :":dbl, element #7=→"AMB_T :":dbl, element #8=→"PUMP :":dbl, element #9=→"FAN_IN :":dbl, element #10=→"FAN_OUT :":dbl, element #11=→"DEHUM :":dbl, element #12=→"CURRENT :":dbl, element #13=→"STALL":dbl)  [unwired: 13 in]
        "RH Numeric:" <- w4440
        n3380 = Equal?(x=w4440, y=0.0) -> (x = y?=w4443:bool)
        n3381 = case shown="False" w4443 {
          tunnel: [w4461 w4462] -> w4444
          tunnel: w4440 -> [w4461 _]
          frame False {
            "Humidity temp 2" <- w4461
          }
          frame True {
            n3382 = local read "Humidity temp 2"() -> (w4462:dbl)
          }
        }
        n3383 = local write "RH Numeric:"(w4444) -> ()
      }
    }
    n3384 = local read "Quit"() -> (w4410:bool)
  }
  n3385 = while {
    shift-right: [w4468] -> _
    shift-left: _ -> [w4469]
    shift-right: [w4466] -> _
    shift-left: T20 {"Read Uno"="", "Bytes at Heave Port"=0.0, "UNO COM Port:"="COM9", "UNO COM Port: 2"="COM7", "Residual Due"="", "UNO COM Status 2"=TRUE, "UNO COM Status"=TRUE, "Port 2"=TRUE, "Sway PPR"=6400.0, "Surge PPR"=6400.0, "Heave PPR"=6400.0, "Sway Pitch"=2.0, "Surge Pitch"=3.0, "Heave Pitch"=4.0, "Sway Pulses/mm"=320.0, "Surge Pulses/mm"=1600.0, "Heave Pulses/mm"=1600.0, "inner loop"=0.0, "Read Heave and Surge 2"="", "String 36"="", "Write S"=FALSE, "WriteCC1"=[""], "Heave COM Loop"=0, "LastCom"="", "EXIT"=FALSE, "Error Heave"={"status"=TRUE, "code"=-1073807343, "source"=""}} -> [w4465]
    shift-right: [w4463] -> _
    shift-left: enum16{"init", "MAIN", "Panel Close"}."init" -> [w4464]
    stop <- w4467 stop-if-true
    # "UNO CODE LOGIC"
    n3386 = case shown="\"MAIN\"" w4464 {
      tunnel: w4469 -> [w4483 w4502 w4558 w4560]
      tunnel: [w4478 w4507 w4558 w4560] -> w4468
      tunnel: [_ _ TRUE _] -> w4467
      tunnel: [w4474 w4505 w4556 w4559] -> w4466
      tunnel: w4465 -> [w4480 w4501 w4556 w4559]
      tunnel: [enum16{"init", "MAIN", "Panel Close"}."MAIN" w4496 _ _] -> w4463
      frame "init" {
        n3387 = local read "Com Port 1"() -> (w4470:refnum<visa-resource-name>)
        n3388 = Bundle By Name(cluster=w4480, "UNO COM Port:"=w4470) -> (w4479:T20)
        n3389 = call "Instrument fgv.vi"("Enum"=T32."INIT", "error in (no error) 2"=w4483, "INPUT"=w4479) -> ("error"=w4481:errorcluster, "output"=w4477:T18)  [unwired: 6 in, 1 out]
        n3390 = case shown="Error" w4481 {
          selector: w4481 -> [w4485 _]
          tunnel: [w4485 w4489] -> w4478
          tunnel: w4477 -> [w4484 w4487]
          tunnel: [w4484 w4486] -> w4475
          frame No Error {
          }
          frame Error {
            n3391 = call "Instrument fgv.vi"("Enum"=T32."ERROR INIT", "INPUT"=w4487) -> ("error"=w4490:errorcluster, "output"=w4486:T18)  [unwired: 7 in, 1 out]
            n3392 = call <vilib>:"Clear Errors.vi"("error in (no error)"=w4490) -> ("error out"=w4489:errorcluster)  [unwired: 5 in, 1 out]
          }
        }
        n3393 = local read "LastCom UNO"() -> (w4472:string)
        n3394 = Unbundle By Name(w4475) -> ("Heave COM Status 2"=→"Instrument Status":bool, "Error Heave"=→"Error  2":errorcluster)  [unwired: 1 out]
        n3395 = Bundle By Name(cluster=w4475, "LastCom"=w4472) -> (w4474:T18)
      }
      frame "MAIN" {
        n3396 = Unbundle By Name(w4501) -> ("UNO COM Port: 2"=w4491:refnum<visa-resource-name>)
        n3397 = local read "Com Port 1"() -> (w4492:refnum<visa-resource-name>)
        n3398 = local write "COM Port UNO :"(w4491) -> ()
        n3399 = Equal?(x=w4491, y=w4492) -> (x = y?=w4508:bool)
        n3400 = Bundle By Name(cluster=w4501, "UNO COM Port:"=w4492) -> (w4500:T20)
        n3401 = case shown="True" w4508 {
          tunnel: [w4512 w4529] -> w4507
          tunnel: w4502 -> [w4513 w4535]
          tunnel: w4500 -> [w4511 w4533]
          tunnel: [w4510 w4528] -> w4505
          frame False {
            n3402 = call <vilib>:"Clear Errors.vi"("error in (no error)"=w4513) -> ("error out"=w4509:errorcluster)  [unwired: 5 in, 1 out]
            n3403 = call "Instrument fgv.vi"("Enum"=T32."ERROR INIT", "error in (no error) 2"=w4509, "INPUT"=w4511) -> ("error"=w4515:errorcluster, "output"=w4510:T18)  [unwired: 6 in, 1 out]
            n3404 = call <vilib>:"Clear Errors.vi"("error in (no error)"=w4515) -> ("error out"=w4512:errorcluster)  [unwired: 5 in, 1 out]
          }
          frame True {
            n3405 = call "Instrument fgv.vi"("Enum"=T32."READ", "error in (no error) 2"=w4535, "INPUT"=w4533) -> ("error"=w4534:errorcluster, "output"=w4527:T18)  [unwired: 6 in, 1 out]
            n3406 = Bundle By Name(cluster=w4527, "String 36"="WRITE UNO") -> (w4526:T18)
            n3407 = case shown="True" "Write" {
              selector: "Write" -> [_ w4550]
              tunnel: w4534 -> [w4548 w4555]
              tunnel: [w4548 w4554] -> w4524
              tunnel: w4526 -> [w4547 w4552]
              tunnel: [w4547 w4551] -> w4523
              frame False {
              }
              frame True {
                n3408 = Not(x=w4550) -> (.not. x?=w4549:bool)
                n3409 = local write "Write"(w4549) -> ()
                n3410 = call "Instrument fgv.vi"("Enum"=T32."MANUAL WRITE", "error in (no error) 2"=w4555, "INPUT"=w4552) -> ("error"=w4554:errorcluster, "output"=w4551:T18)  [unwired: 6 in, 1 out]
              }
            }
            n3411 = Array Size(array="Write UNO") -> (size(s)=w4521:i32)
            n3412 = Greater Than 0?(x=w4521) -> (x > 0?=w4520:bool)
            n3413 = call "Instrument fgv.vi"("Enum"=T32."WRITE", "error in (no error) 2"=w4524, "WriteCC1"="Write UNO", "INPUT"=w4523) -> ("error"=w4531:errorcluster, "WriteCC1 2"=w4522:string[], "output"=w4530:T18)  [unwired: 5 in]
            n3414 = case shown="True" w4520 {
              tunnel: w4522 -> [_ w4537]
              frame False {
              }
              frame True {
                n3415 = local write "Write UNO"(w4537) -> ()
              }
            }
            n3416 = case shown="Error" w4531 {
              selector: w4531 -> [w4538 w4541]
              tunnel: w4530 -> [w4539 w4546]
              tunnel: [w4539 w4545] -> w4528
              tunnel: [w4538 w4543] -> w4529
              frame No Error {
              }
              frame Error {
                n3417 = call <vilib>:"Clear Errors.vi"("error in (no error)"=w4541) -> ("error out"=w4540:errorcluster)  [unwired: 5 in, 1 out]
                n3418 = call "Instrument fgv.vi"("Enum"=T32."ERROR INIT", "error in (no error) 2"=w4540, "INPUT"=w4546) -> ("error"=w4544:errorcluster, "output"=w4545:T18)  [unwired: 6 in, 1 out]
                n3419 = call <vilib>:"Clear Errors.vi"("error in (no error)"=w4544) -> ("error out"=w4543:errorcluster)  [unwired: 5 in, 1 out]
              }
            }
            n3420 = Unbundle By Name(w4528) -> ("LastCom"=→"LastCom UNO":string, "Read Heave and Surge"=→"Read UNO":string)
          }
        }
        n3421 = Unbundle By Name(w4505) -> ("Heave COM Status 2"=w4506:bool, "Heave COM Status"=w4495:bool, "Error Heave"=w4493:errorcluster, "Bytes at Heave Port"=→"Bytes at Humidity Port":dbl)
        n3422 = Not(x=w4495) -> (.not. x?=w4503:bool)
        n3423 = Not(x=w4506) -> (.not. x?=w4494:bool)
        n3424 = local write "Instrument Status"(w4503) -> ()
        n3425 = local write "Error  2"(w4493) -> ()
        n3426 = local write "Port 1a"(w4495) -> ()
        n3427 = local read "Quit"() -> (w4497:bool)
        n3428 = local write "COM Status"(w4494) -> ()
        n3429 = Select(t=enum16{"init", "MAIN", "Panel Close"}."Panel Close", s=w4497, f=enum16{"init", "MAIN", "Panel Close"}."MAIN") -> (s? t:f=w4496:enum16{"init", "MAIN", "Panel Close"})
      }
      frame "Panel Close" {
      }
      frame Default {
      }
    }
  }
